vi "Capture Audio (Polymorphic Template).vi"   [LabVIEW 2020]
uses:
  563bab1f-8f2c-4ac6-9d66-29acee9d0e05.vi
  8efdc9b5-88b6-4924-8582-0cb5cfe414ea.vi
  a9e01df1-edab-454f-b888-4afc9940cde3.vi
  0cb032c8-6079-43b3-be5d-cda8a1799209.vi
  cde89a8b-461d-453a-904f-53541ab8ccbd.vi
  234c1178-5d48-43e8-a738-60ddbd5433f2.vi
  53b3f6ff-4d26-4a4a-a60b-69c08edf7529.vi
  5bf22e26-9c1f-4502-867f-b9a33ff147b8.vi
  b44b48c6-dc6a-41e8-ad0f-ee80fd1b0c25.vi
  506ae791-0beb-420c-bcfe-c42f9d99f998.vi
  748d3671-1ea6-4799-8456-0925c563e01a.vi
  351f5817-6162-4094-abf3-5b2ac090c9e6.vi
  fed51032-3ea9-4983-a892-1122525d9d24.vi
  96d6df5f-e3cb-4a5f-94cb-bcb3fc8a759d.vi
  b97cbd95-6807-468a-9906-0abf1bdbe7e9.vi
  86932fcd-11a2-404e-a7ec-91da0a9d7749.vi
  7fcb6284-5da8-4912-8687-27a442e8dfad.vi
  ca60281f-2b22-4b8a-8ed8-e3e9c614b86b.vi
  6d8c1217-7206-47a1-8c68-00e96129c59b.vi
  f8af4853-b22c-49db-ae14-7d8402abbb96.vi
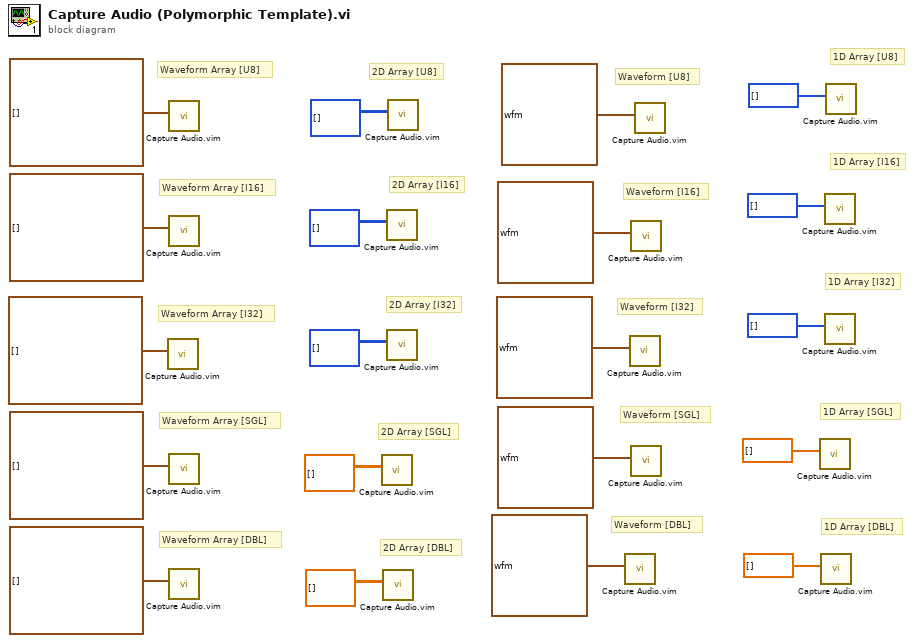
[diagram p0: block diagram]
diagram:
  # "1D Array [DBL]"
  # "1D Array [SGL]"
  # "1D Array [I32]"
  # "1D Array [I16]"
  # "1D Array [U8]"
  # "Waveform [DBL]"
  # "Waveform [SGL]"
  # "Waveform [I32]"
  # "Waveform [I16]"
  # "Waveform [U8]"
  # "2D Array [DBL]"
  # "2D Array [SGL]"
  # "2D Array [I32]"
  # "2D Array [I16]"
  # "2D Array [U8]"
  # "Waveform Array [DBL]"
  # "Waveform Array [SGL]"
  # "Waveform Array [I32]"
  # "Waveform Array [I16]"
  # "Waveform Array [U8]"
  n1 = call "Capture Audio.vim"("Data Format"=waveform(i32)[] [] ("Data Format (I16 Waveform Array)")) -> ()  [unwired: 8 in, 3 out]
  n2 = call "Capture Audio.vim"("Data Format"=waveform(u8)[] [] ("Data Format (I16 Waveform Array)")) -> ()  [unwired: 8 in, 3 out]
  n3 = call "Capture Audio.vim"("Data Format"=waveform(i16)[] [] ("Data Format (I16 Waveform Array)")) -> ()  [unwired: 8 in, 3 out]
  n4 = call "Capture Audio.vim"("Data Format"=waveform(sgl)[] [] ("Data Format (I16 Waveform Array)")) -> ()  [unwired: 8 in, 3 out]
  n5 = call "Capture Audio.vim"("Data Format"=waveform(dbl)[] [] ("Data Format (I16 Waveform Array)")) -> ()  [unwired: 8 in, 3 out]
  n6 = call "Capture Audio.vim"("Data Format"=sgl[][] []) -> ()  [unwired: 8 in, 3 out]
  n7 = call "Capture Audio.vim"("Data Format"=dbl[][] []) -> ()  [unwired: 8 in, 3 out]
  n8 = call "Capture Audio.vim"("Data Format"=i16[][] []) -> ()  [unwired: 8 in, 3 out]
  n9 = call "Capture Audio.vim"("Data Format"=i32[][] []) -> ()  [unwired: 8 in, 3 out]
  n10 = call "Capture Audio.vim"("Data Format"=u8[][] []) -> ()  [unwired: 8 in, 3 out]
  n11 = call "Capture Audio.vim"("Data Format"=waveform(dbl) {"t0"=timestamp(0 s since 1904-01-01), "dt"=1.0, "Y"=[]} ("Waveform")) -> ()  [unwired: 8 in, 3 out]
  n12 = call "Capture Audio.vim"("Data Format"=waveform(i32) {"t0"=timestamp(0 s since 1904-01-01), "dt"=1.0, "Y"=[]} ("Waveform")) -> ()  [unwired: 8 in, 3 out]
  n13 = call "Capture Audio.vim"("Data Format"=waveform(i16) {"t0"=timestamp(0 s since 1904-01-01), "dt"=1.0, "Y"=[]} ("Waveform")) -> ()  [unwired: 8 in, 3 out]
  n14 = call "Capture Audio.vim"("Data Format"=waveform(sgl) {"t0"=timestamp(0 s since 1904-01-01), "dt"=1.0, "Y"=[]} ("Waveform")) -> ()  [unwired: 8 in, 3 out]
  n15 = call "Capture Audio.vim"("Data Format"=waveform(u8) {"t0"=timestamp(0 s since 1904-01-01), "dt"=1.0, "Y"=[]} ("Waveform")) -> ()  [unwired: 8 in, 3 out]
  n16 = call "Capture Audio.vim"("Data Format"=sgl[] []) -> ()  [unwired: 8 in, 3 out]
  n17 = call "Capture Audio.vim"("Data Format"=dbl[] []) -> ()  [unwired: 8 in, 3 out]
  n18 = call "Capture Audio.vim"("Data Format"=i16[] []) -> ()  [unwired: 8 in, 3 out]
  n19 = call "Capture Audio.vim"("Data Format"=i32[] []) -> ()  [unwired: 8 in, 3 out]
  n20 = call "Capture Audio.vim"("Data Format"=u8[] []) -> ()  [unwired: 8 in, 3 out]
